vi "15-12-13 UHR-Fleezers Control (host) - 15.2.1UCB Darwin.vi"() -> ()   [LabVIEW 2014] (continued)
        n372 = stacked-sequence {
          tunnel: [w623] -> w618
          tunnel: w620 -> [w623]
          tunnel: w619 -> [w622]
          tunnel: [w622] -> w613
          frame #0 {
            n373 = Wait (ms)(milliseconds to wait=50) -> ()  [unwired: 1 out]
          }
        }
        n374 = property class="Instr"(reference=w618, error in=w613) -> (reference out=w617:refnum<visa-resource-name>, error out=w615:errorcluster, "Serial Settings:Number of Bytes at Serial Port"=w616:u32)
        "Serial Settings:Number of Bytes at Serial Port" <- w616
        n375 = VISA Read(VISA resource name=w617, byte count=w616, error in (no error)=w615) -> (read buffer=w614:string)  [unwired: 3 out]
        "read buffer" <- w614
        n376 = Fract/Exp String To Number(string=w614) -> ()  [unwired: 5 out]
      }
      event "+z", "-z": Value Change {
        n377 = event-data() -> ()  [unwired: 1 in, 5 out]
        n378 = flat-sequence {
          tunnel: w624 -> [w646]
          tunnel: w625 -> [w626]
          frame #0 {
            n379 = call "Read Stage Position.vi"("error in"=w646, "VISA resource name in"=w626) -> ("Current Position"=w631:cluster{dbl, dbl, dbl}, "error out"=w644:errorcluster, "VISA resource name out"=w645:refnum<visa-resource-name>)  [unwired: 1 out]
            n380 = local read "Saved Stage Positions"() -> (w655:dbl[][])
            n381 = Divide(x="z nudge increment (um)", y=1000.0) -> (x/y=w643:dbl)
            n382 = Boolean To (0,1)(Boolean="+z") -> (0, 1=w635:i16)
            n383 = Boolean To (0,1)(Boolean="-z") -> (0, 1=w636:i16)
            n384 = Array Subset(array=w655, index (row)=1 ("index"), length (row)=1 ("length"), index (col)=1 ("index"), length (col)=3 ("length")) -> (w652:dbl[][])
            n385 = Multiply(x=w635, y=w643) -> (x*y=w639:dbl)
            n386 = Multiply(x=w636, y=w643) -> (x*y=w637:dbl)
            n387 = Unbundle(w631) -> (w629:dbl, w628:dbl, w632:dbl)
            n388 = Negate(x=w637) -> (-x=w638:dbl)
            n389 = Reshape Array(w652, 3 ("dimension size")) -> (w650:dbl[])
            n390 = Add(x=w639, y=w638) -> (x+y=w640:dbl)
            n391 = Array To Cluster(array=w650) -> ()  [unwired: 1 out]
            n392 = Add(x=w640, y=w632) -> (x+y=w630:dbl)
            n393 = Bundle(cluster=w631, w629, w628, w630) -> (w627:cluster{dbl, dbl, dbl})
            n394 = call "Set Stage Position.vi"("Position"=w627, "error in"=w644, "VISA resource name in"=w645) -> ("error out"=w649:errorcluster)  [unwired: 2 out]
            n395 = local write "Stage Moving"(TRUE ("Stage Moving")) -> ()
            n396 = local write "Stage Control Serial Error"(w649) -> ()
          }
          frame #1 {
            n397 = local write "Stage Moving"(FALSE ("Stage Moving")) -> ()
          }
        }
      }
      event "-y", "+y": Value Change {
        n398 = event-data() -> ()  [unwired: 1 in, 5 out]
        n399 = flat-sequence {
          tunnel: w658 -> [w682]
          tunnel: w659 -> [w665]
          frame #0 {
            n400 = call "Read Stage Position.vi"("error in"=w682, "VISA resource name in"=w665) -> ("Current Position"=w668:cluster{dbl, dbl, dbl}, "error out"=w680:errorcluster, "VISA resource name out"=w681:refnum<visa-resource-name>)  [unwired: 1 out]
            n401 = Divide(x="y nudge increment (um", y=1000.0) -> (x/y=w679:dbl)
            n402 = Boolean To (0,1)(Boolean="+y") -> (0, 1=w671:i16)
            n403 = Boolean To (0,1)(Boolean="-y") -> (0, 1=w672:i16)
            n404 = Multiply(x=w671, y=w679) -> (x*y=w675:dbl)
            n405 = Multiply(x=w672, y=w679) -> (x*y=w673:dbl)
            n406 = Unbundle(w668) -> (w667:dbl, w662:dbl, w664:dbl)
            n407 = Negate(x=w673) -> (-x=w674:dbl)
            n408 = Add(x=w675, y=w674) -> (x+y=w676:dbl)
            n409 = Add(x=w676, y=w662) -> (x+y=w663:dbl)
            n410 = Bundle(cluster=w668, w667, w663, w664) -> (w666:cluster{dbl, dbl, dbl})
            n411 = call "Set Stage Position.vi"("Position"=w666, "error in"=w680, "VISA resource name in"=w681) -> ("error out"=w661:errorcluster)  [unwired: 2 out]
            n412 = local write "Stage Control Serial Error"(w661) -> ()
            n413 = local write "Stage Moving"(TRUE ("Stage Moving")) -> ()
          }
          frame #1 {
            n414 = local write "Stage Moving"(FALSE ("Stage Moving")) -> ()
          }
        }
      }
      event "-x", "+x": Value Change {
        n415 = event-data() -> ()  [unwired: 1 in, 5 out]
        n416 = flat-sequence {
          tunnel: w684 -> [w708]
          tunnel: w685 -> [w692]
          frame #0 {
            n417 = call "Read Stage Position.vi"("error in"=w708, "VISA resource name in"=w692) -> ("Current Position"=w694:cluster{dbl, dbl, dbl}, "error out"=w706:errorcluster, "VISA resource name out"=w707:refnum<visa-resource-name>)  [unwired: 1 out]
            n418 = Divide(x="x nudge increment (um)", y=1000.0) -> (x/y=w705:dbl)
            n419 = Boolean To (0,1)(Boolean="+x") -> (0, 1=w697:i16)
            n420 = Boolean To (0,1)(Boolean="-x") -> (0, 1=w698:i16)
            n421 = Multiply(x=w697, y=w705) -> (x*y=w701:dbl)
            n422 = Multiply(x=w698, y=w705) -> (x*y=w699:dbl)
            n423 = Unbundle(w694) -> (w686:dbl, w688:dbl, w691:dbl)
            n424 = Negate(x=w699) -> (-x=w700:dbl)
            n425 = Add(x=w701, y=w700) -> (x+y=w702:dbl)
            n426 = Add(x=w702, y=w686) -> (x+y=w687:dbl)
            n427 = Bundle(cluster=w694, w687, w688, w691) -> (w693:cluster{dbl, dbl, dbl})
            n428 = call "Set Stage Position.vi"("Position"=w693, "error in"=w706, "VISA resource name in"=w707) -> ("error out"=w689:errorcluster)  [unwired: 2 out]
            n429 = local write "Stage Control Serial Error"(w689) -> ()
            n430 = local write "Stage Moving"(TRUE ("Stage Moving")) -> ()
          }
          frame #1 {
            n431 = local write "Stage Moving"(FALSE ("Stage Moving")) -> ()
          }
        }
      }
      event "Cal/Data Acq. Spot": Value Change {
        n432 = event-data() -> ()  [unwired: 1 in, 5 out]
        n433 = flat-sequence {
          tunnel: w716 -> [w720]
          tunnel: w717 -> [w721]
          tunnel: [w721] -> w713
          tunnel: [w720] -> w712
          tunnel: w713 -> [w726]
          tunnel: w712 -> [w725]
          tunnel: ["Cal @ (MHz)"] -> w710
          tunnel: [w730] -> w714
          tunnel: w710 -> [w730]
          tunnel: w714 -> [w742]
          tunnel: ["W/ Offset 1"] -> w711
          tunnel: w714 -> [w763]
          tunnel: w711 -> [w761]
          frame #0 {
            n434 = property on="Sample Channel\nFlow" class="Bool (strict)"("Val(Sgnl)"="Daq spot flow on") -> ()  [unwired: 2 in, 2 out]
            n435 = Wait (ms)(milliseconds to wait=u32 250) -> ()  [unwired: 1 out]
          }
          frame #1 {
            n436 = local read "Saved Stage Positions"() -> (w723:dbl[][])
            n437 = property on="Trap Delta (MHz)" class="DigNum (strict)"("Val(Sgnl)"="Cal @ (MHz)") -> ()  [unwired: 2 in, 2 out]
            n438 = local write "Stage Moving"(TRUE ("Stage Moving")) -> ()
            n439 = call "move to saved stage position.vi"("error in"=w725, "Stage VISA resource name in"=w726, "Position"="Cal Stage Position", "Saved Stage Positions"=w723) -> ("error out"=w724:errorcluster)  [unwired: 1 out]
            n440 = local write "Stage Control Serial Error"(w724) -> ()
          }
          frame #2 {
            n441 = local write "Stage Moving"(FALSE ("Stage Moving")) -> ()
            n442 = property on="Sample Channel\nFlow" class="Bool (strict)"("Val(Sgnl)"="Flow ON during cal?") -> ()  [unwired: 2 in, 2 out]
            n443 = call <vilib>:"Beep.vi"() -> ()  [unwired: 3 in, 9 out]
          }
          frame #3 {
            n444 = Wait (ms)(milliseconds to wait=u32 1000) -> ()  [unwired: 1 out]
          }
          frame #4 {
            n445 = case shown="True" "Active cal after cal?" {
              frame False {
              }
              frame True {
                n446 = local write "Active Cal"(TRUE ("Active Cal")) -> ()
                n447 = Wait (ms)(milliseconds to wait=u32 8000) -> ()  [unwired: 1 out]
              }
            }
          }
          frame #5 {
            n448 = property on="Save Calibration" class="Bool (strict)"("Val(Sgnl)"=TRUE ("Value (Signaling)")) -> ()  [unwired: 2 in, 2 out]
          }
          frame #6 {
            n449 = Wait (ms)(milliseconds to wait=u32 2000) -> ()  [unwired: 1 out]
          }
          frame #7 {
            # "Check to see if \nsaving done"
            n450 = while {
              stop <- w738 stop-if-true
              n451 = local read "Saving..."() -> (w739:bool)
              n452 = Wait (ms)(milliseconds to wait=u32 100) -> ()  [unwired: 1 out]
              n453 = Not(x=w739) -> (.not. x?=w738:bool)
            }
          }
          frame #8 {
            n454 = case shown="True" "W/ Offset 1" {
              tunnel: w742 -> [_ w743]
              frame False {
              }
              frame True {
                n455 = stacked-sequence {
                  tunnel: w743 -> [_ _ _ _ _ _ _ w760]
                  frame #0 {
                    n456 = property on="Trap Delta (MHz)" class="DigNum (strict)"("Val(Sgnl)"="Offset 1 Start (MHz)") -> ()  [unwired: 2 in, 2 out]
                    n457 = Replace Array Subset(array=u32[] [0] ("Index Values"), new element="Offset 1 Set", index=0) -> (w744:u32[])
                    n458 = property on="Saved AOD Raster Scan Parameter Sets" class="Arr (strict)"("Index Values"=w744) -> ()  [unwired: 2 in, 2 out]
                  }
                  frame #1 {
                    n459 = Wait (ms)(milliseconds to wait=u32 200) -> ()  [unwired: 1 out]
                  }
                  frame #2 {
                    n460 = property on="Load parameters" class="Bool (strict)"("Val(Sgnl)"=TRUE ("Value (Signaling)")) -> ()  [unwired: 2 in, 2 out]
                  }
                  frame #3 {
                    n461 = Wait (ms)(milliseconds to wait=u32 200) -> ()  [unwired: 1 out]
                  }
                  frame #4 {
                    n462 = property on="Trap Raster Scan" class="Bool (strict)"("Val(Sgnl)"=TRUE ("Value (Signaling)")) -> ()  [unwired: 2 in, 2 out]
                  }
                  frame #5 {
                    n463 = Wait (ms)(milliseconds to wait=u32 2000) -> ()  [unwired: 1 out]
                  }
                  frame #6 {
                    n464 = while {
                      stop <- w757 stop-if-true
                      n465 = local read "Raster Scanning..."() -> (w759:bool)
                      n466 = local read "Saving..."() -> (w755:bool)
                      n467 = Wait (ms)(milliseconds to wait=u32 100) -> ()  [unwired: 1 out]
                      n468 = Not(x=w755) -> (.not. x?=w754:bool)
                      n469 = Not(x=w759) -> (.not. x?=w756:bool)
                      n470 = And(x=w756, y=w754) -> (x .and. y?=w757:bool)
                    }
                  }
                  frame #7 {
                    n471 = property on="Trap Delta (MHz)" class="DigNum (strict)"("Val(Sgnl)"=w760) -> ()  [unwired: 2 in, 2 out]
                  }
                }
              }
            }
          }
          frame #9 {
            n472 = local read "Save ave N"() -> (w762:dbl)
            n473 = case shown="False" "W/ Offset 2" {
              tunnel: w763 -> [_ w770]
              tunnel: w762 -> [_ w769]
              tunnel: w761 -> [w765 _]
              frame False {
                n474 = case shown="False" w765 {
                  frame False {
                    n475 = Multiply(x="Cal read wait (s)", y=u32 1000 ("milliseconds to wait")) -> (x*y=w767:u32)
                    n476 = Wait (ms)(milliseconds to wait=w767) -> ()  [unwired: 1 out]
                  }
                  frame True {
                  }
                }
              }
              frame True {
                n477 = stacked-sequence {
                  tunnel: w770 -> [_ _ _ _ _ _ _ _ _ w791 _ _]
                  tunnel: w769 -> [_ _ _ _ _ _ _ _ _ w789 _ _]
                  frame #0 {
                    n478 = property on="Save ave N" class="DigNum (strict)"("Val(Sgnl)"=1.0 ("Value (Signaling)")) -> ()  [unwired: 2 in, 2 out]
                  }
                  frame #1 {
                    n479 = Wait (ms)(milliseconds to wait=u32 500) -> ()  [unwired: 1 out]
                  }
                  frame #2 {
                    n480 = property on="Trap Delta (MHz)" class="DigNum (strict)"("Val(Sgnl)"="Offset 2 Start (MHz)") -> ()  [unwired: 2 in, 2 out]
                    n481 = Replace Array Subset(array=u32[] [0] ("Index Values"), new element="Offset 2 Set", index=0) -> (w775:u32[])
                    n482 = property on="Saved AOD Raster Scan Parameter Sets" class="Arr (strict)"("Index Values"=w775) -> ()  [unwired: 2 in, 2 out]
                  }
                  frame #3 {
                    n483 = Wait (ms)(milliseconds to wait=u32 500) -> ()  [unwired: 1 out]
                  }
                  frame #4 {
                    n484 = property on="Load parameters" class="Bool (strict)"("Val(Sgnl)"=TRUE ("Value (Signaling)")) -> ()  [unwired: 2 in, 2 out]
                  }
                  frame #5 {
                    n485 = Wait (ms)(milliseconds to wait=u32 500) -> ()  [unwired: 1 out]
                  }
                  frame #6 {
                    n486 = property on="Trap Raster Scan" class="Bool (strict)"("Val(Sgnl)"=TRUE ("Value (Signaling)")) -> ()  [unwired: 2 in, 2 out]
                  }
                  frame #7 {
                    n487 = Wait (ms)(milliseconds to wait=u32 2000) -> ()  [unwired: 1 out]
                  }
                  frame #8 {
                    n488 = while {
                      stop <- w784 stop-if-true
                      n489 = local read "Raster Scanning..."() -> (w787:bool)
                      n490 = local read "Saving..."() -> (w785:bool)
                      n491 = Wait (ms)(milliseconds to wait=u32 100) -> ()  [unwired: 1 out]
                      n492 = Not(x=w785) -> (.not. x?=w783:bool)
                      n493 = Not(x=w787) -> (.not. x?=w786:bool)
                      n494 = And(x=w786, y=w783) -> (x .and. y?=w784:bool)
                    }
                  }
                  frame #9 {
                    n495 = property on="Trap Delta (MHz)" class="DigNum (strict)"("Val(Sgnl)"=w791) -> ()  [unwired: 2 in, 2 out]
                    n496 = property on="Saved AOD Raster Scan Parameter Sets" class="Arr (strict)"("Index Values"=u32[] [0]) -> ()  [unwired: 2 in, 2 out]
                    n497 = property on="Save ave N" class="DigNum (strict)"("Val(Sgnl)"=w789) -> ()  [unwired: 2 in, 2 out]
                  }
                  frame #10 {
                    n498 = Wait (ms)(milliseconds to wait=u32 500) -> ()  [unwired: 1 out]
                  }
                  frame #11 {
                    n499 = property on="Load parameters" class="Bool (strict)"("Val(Sgnl)"=TRUE ("Value (Signaling)")) -> ()  [unwired: 2 in, 2 out]
                  }
                }
              }
            }
          }
          frame #10 {
            n500 = property on="Read Cal" class="Bool (strict)"("Val(Sgnl)"=TRUE ("Value (Signaling)")) -> ()  [unwired: 2 in, 2 out]
          }
          frame #11 {
            n501 = Wait (ms)(milliseconds to wait=u32 1000) -> ()  [unwired: 1 out]
          }
          frame #12 {
            n502 = property on="Fish for Tether" class="Bool (strict)"("Val(Sgnl)"="Fish after cal?") -> ()  [unwired: 2 in, 2 out]
          }
        }
        n503 = local write "Cal/Data Acq. Spot"(FALSE ("Cal/Data Acq. Spot")) -> ()
      }
      event "Dump Beads": Value Change {
        n504 = event-data() -> ()  [unwired: 1 in, 5 out]
        n505 = flat-sequence {
          tunnel: ["Dump spot flow on?"] -> w797
          tunnel: [w808] -> w798
          tunnel: w797 -> [w808]
          tunnel: w801 -> [w813]
          tunnel: w800 -> [w812]
          tunnel: [w810] -> w799
          tunnel: w798 -> [w810]
          tunnel: w799 -> [w823]
          frame #0 {
            w802 = FALSE ("Value (Signaling)")
            n506 = local read "Saving..."() -> (w804:bool)
            n507 = local write "Dump Beads"(FALSE ("Dump Beads")) -> ()
            n508 = property on="Inject Pump 3" class="Bool (strict)"("Val(Sgnl)"=w802) -> ()  [unwired: 2 in, 2 out]
            n509 = property on="Inject Pump 1" class="Bool (strict)"("Val(Sgnl)"=w802) -> ()  [unwired: 2 in, 2 out]
            n510 = local write "Stop Saving"(w804) -> ()
          }
          frame #1 {
            w805 = FALSE ("Fl. Triggered...")
            n511 = case shown="True" "Dump spot flow on?" {
              frame False {
              }
              frame True {
                n512 = property on="Sample Channel\nFlow" class="Bool (strict)"("Val(Sgnl)"=TRUE ("Stage Moving")) -> ()  [unwired: 2 in, 2 out]
              }
            }
            n513 = local write "Fl. Triggered..."(w805) -> ()
            n514 = local write "Tether"(w805) -> ()
            n515 = property on="Green Laser ON" class="Bool (strict)"("Val(Sgnl)"=w805) -> ()  [unwired: 2 in, 2 out]
            n516 = property on="Trap Pos. FB ON" class="Bool (strict)"("Val(Sgnl)"=w805) -> ()  [unwired: 2 in, 2 out]
            n517 = property on="Trap Trig. Fl." class="Bool (strict)"("Val(Sgnl)"=w805) -> ()  [unwired: 2 in, 2 out]
            n518 = property on="Fl. Triggered..." class="Bool (strict)"("Val(Sgnl)"=w805) -> ()  [unwired: 2 in, 2 out]
            n519 = property on="Dip for Protein" class="Bool (strict)"("Val(Sgnl)"=w805) -> ()  [unwired: 2 in, 2 out]
            n520 = property on="Pause dwell" class="Bool (strict)"("Val(Sgnl)"=w805) -> ()  [unwired: 2 in, 2 out]
          }
          frame #2 {
            n521 = property on="Trap Pos. FB Offset Factor" class="DigNum (strict)"("Val(Sgnl)"=i64 0 ("Value (Signaling)")) -> ()  [unwired: 2 in, 2 out]
          }
          frame #3 {
            n522 = local read "Saved Stage Positions"() -> (w814:dbl[][])
            n523 = local write "Stage Moving"(TRUE ("Stage Moving")) -> ()
            n524 = Array Subset(array=w814, index (row)=3 ("index"), length (row)=1 ("length"), index (col)=1 ("index"), length (col)=3 ("length")) -> (w819:dbl[][])
            n525 = Reshape Array(w819, 3 ("dimension size")) -> (w817:dbl[])
            n526 = Array To Cluster(array=w817) -> (cluster=w816:cluster{"[0]":dbl, "[1]":dbl, "[2]":dbl})
            n527 = call "Set Stage Position.vi"("Position"=w816, "error in"=w812, "VISA resource name in"=w813) -> ()  [unwired: 3 out]
          }
          frame #4 {
            w824 = FALSE ("Value (Signaling)")
            n528 = case shown="True" w823 {
              frame False {
              }
              frame True {
                n529 = property on="Sample Channel\nFlow" class="Bool (strict)"("Val(Sgnl)"=FALSE ("Stage Moving")) -> ()  [unwired: 2 in, 2 out]
              }
            }
            n530 = property on="Trap 1 (ON/OFF)" class="Bool (strict)"("Val(Sgnl)"=w824) -> ()  [unwired: 2 in, 2 out]
            n531 = property on="Trap 2 (ON/OFF)" class="Bool (strict)"("Val(Sgnl)"=w824) -> ()  [unwired: 2 in, 2 out]
            n532 = call <vilib>:"Beep.vi"() -> ()  [unwired: 3 in, 9 out]
          }
          frame #5 {
            n533 = property on="Move Cap. 2 (ADig Top)" class="Bool (strict)"("Val(Sgnl)"=TRUE ("Value (Signaling)")) -> ()  [unwired: 2 in, 2 out]
            n534 = property on="Tab Control" class="TabCtl (strict)"("Val(Sgnl)"=T30."Status" ("Value (Signaling)")) -> ()  [unwired: 2 in, 2 out]
          }
        }
      }
      event "Dip for Protein": Value Change {
        n535 = event-data() -> ()  [unwired: 1 in, 5 out]
        n536 = case shown="True" "Dip for Protein" {
          tunnel: w830 -> [_ w832]
          tunnel: w829 -> [_ w831]
          frame False {
          }
          frame True {
            n537 = while {
              tunnel: w832 -> [w843]
              tunnel: w831 -> [w842]
              i -> [w837]
              stop <- w839 stop-if-true
              n538 = Increment(x=w837) -> (x+1=→"Dip #":i32)
              n539 = flat-sequence {
                tunnel: w842 -> [w854]
                tunnel: w843 -> [w855]
                tunnel: [w855] -> w847
                tunnel: [w854] -> w846
                tunnel: [w848] -> w833
                tunnel: [w860] -> w841
                tunnel: [w861] -> w840
                tunnel: w847 -> [w862]
                tunnel: w846 -> [w863]
                tunnel: [w858] -> w834
                tunnel: w833 -> [w858]
                tunnel: [w871] -> w845
                tunnel: w841 -> [w871]
                tunnel: [w870] -> w844
                tunnel: w840 -> [w870]
                tunnel: [w867] -> w838
                tunnel: [w866] -> w835
                tunnel: w834 -> [w866]
                tunnel: w844 -> [w891]
                tunnel: w845 -> [w892]
                tunnel: w838 -> [w893]
                tunnel: w835 -> [w890]
                tunnel: [w949] -> w839
                frame #0 {
                  n540 = local read "Trap Pos. FB ON"() -> (w848:bool)
                  n541 = Compound Arithmetic op=AND("Flow ON\nduring dip?", "FB OFF when \nflow ON", w848) -> (w849:bool)
                  n542 = case shown="True" "Move trap \nbefore dip move?" {
                    frame False {
                    }
                    frame True {
                      n543 = property on="Trap Delta (MHz)" class="DigNum (strict)"("Val(Sgnl)"="Dipping Delta (MHz)") -> ()  [unwired: 2 in, 2 out]
                    }
                  }
                  n544 = property on="Green Laser ON" class="Bool (strict)"("Val(Sgnl)"="Green ON\nbefore dip?") -> ()  [unwired: 2 in, 2 out]
                  n545 = property on="Sample Channel\nFlow" class="Bool (strict)"("Val(Sgnl)"="Flow ON\nduring dip?") -> ()  [unwired: 2 in, 2 out]
                  n546 = case shown="True" w849 {
                    frame False {
                    }
                    frame True {
                      n547 = property on="Trap Pos. FB ON" class="Bool (strict)"("Val(Sgnl)"=FALSE ("Value (Signaling)")) -> ()  [unwired: 2 in, 2 out]
                    }
                  }
                }
                frame #1 {
                  n548 = local read "Saved Stage Positions"() -> (w865:dbl[][])
                  n549 = local write "Cancel dwell"(FALSE ("Cancel dwell")) -> ()
                  n550 = call "move to saved stage position.vi"("error in"=w863, "Stage VISA resource name in"=w862, "Position"="Dip Stage \nPosition", "Saved Stage Positions"=w865) -> ("VISA resource name out"=w860:refnum<visa-resource-name>, "error out"=w861:errorcluster)
                }
                frame #2 {
                  n551 = node-c288() -> (w869:T27)  [unwired: 4 in]
                  n552 = timed-loop {
                    timing: w869 -> [_]
                    timing-out: [_] -> w868
                    tunnel: [w875] -> w867
                    i -> [w872]
                    stop <- w876 stop-if-true
                    n553 = node-c288() -> ()  [unwired: 1 in, 1 out]
                    n554 = Greater Or Equal?(x=w872, y="Dip Duration (s)") -> (x >= y?=w884:bool)
                    n555 = local read "Dip for Protein"() -> (w877:bool)
                    n556 = local read "Dump Beads"() -> (w874:bool)
                    n557 = local read "Cancel dwell"() -> (w883:bool)
                    n558 = local read "Pause dwell"() -> (w880:bool)
                    n559 = Not(x=w877) -> (.not. x?=w882:bool)
                    n560 = Compound Arithmetic op=OR(w883, w884, w882) -> (w881:bool)
                    n561 = Select(t=FALSE, s=w880, f=w881) -> (s? t:f=w878:bool)
                    n562 = Not(x=w874) -> (.not. x?=w873:bool)
                    n563 = node-c288() -> ()  [unwired: 1 in, 1 out]
                    n564 = And(x=w877, y=w873) -> (x .and. y?=w875:bool)
                    n565 = Or(x=w878, y=w874) -> (x .or. y?=w876:bool)
                    "Dip Time (s)" <- w872
                  }
                  n566 = node-c288(w868) -> ()  [unwired: 1 out]
                }
                frame #3 {
                  n567 = case shown="True" w893 {
                    tunnel: w892 -> [_ w898]
                    tunnel: w891 -> [_ w897]
                    tunnel: w890 -> [_ w894]
                    frame False {
                    }
                    frame True {
                      n568 = flat-sequence {
                        tunnel: w897 -> [w902]
                        tunnel: w898 -> [w903]
                        tunnel: [w903] -> w896
                        tunnel: [w902] -> w895
                        tunnel: w894 -> [w899]
                        tunnel: w896 -> [w913]
                        tunnel: w895 -> [w912]
                        tunnel: w894 -> [w921]
                        frame #0 {
                          n569 = local read "Sample Channel\nFlow"() -> (w901:bool)
                          n570 = case shown="True" w901 {
                            tunnel: "Flow ON \nduring return\nfrom dip?" -> [w904 w907]
                            tunnel: w899 -> [_ w906]
                            frame False {
                              n571 = case shown="True" w904 {
                                frame False {
                                }
                                frame True {
                                n572 = property on="Sample Channel\nFlow" class="Bool (strict)"("Val(Sgnl)"=TRUE ("Value (Signaling)")) -> ()  [unwired: 2 in, 2 out]
                                }
                              }
                            }
                            frame True {
                              n573 = case shown="False" w907 {
                                tunnel: w906 -> [w908 _]
                                frame False {
                                n574 = property on="Trap Pos. FB ON" class="Bool (strict)"("Val(Sgnl)"=w908) -> ()  [unwired: 2 in, 2 out]
                                n575 = property on="Sample Channel\nFlow" class="Bool (strict)"("Val(Sgnl)"=FALSE ("Value (Signaling)")) -> ()  [unwired: 2 in, 2 out]
                                }
                                frame True {
                                }
                              }
                            }
                          }
                        }
                        frame #1 {
                          # "For turning on green laser before stage reaches lower spot"
                          n576 = case shown="True" "Green ON\nafter start\nreturn?" {
                            frame False {
                            }
                            frame True {
                              n577 = flat-sequence {
                                frame #0 {
                                n578 = Multiply(x="Green delay after \nstart return (s)", y=1000.0) -> (x*y=w918:dbl)
                                n579 = Wait (ms)(milliseconds to wait=w918) -> ()  [unwired: 1 out]
                                }
                                frame #1 {
                                n580 = property on="Green Laser ON" class="Bool (strict)"("Val(Sgnl)"=TRUE ("Value (Signaling)")) -> ()  [unwired: 2 in, 2 out]
                                }
                              }
                            }
                          }
                          n581 = local read "Saved Stage Positions"() -> (w916:dbl[][])
                          n582 = local write "Cancel dwell"(FALSE ("Cancel dwell")) -> ()
                          n583 = call "move to saved stage position.vi"("error in"=w912, "Stage VISA resource name in"=w913, "Position"="Return Stage \nPosition", "Saved Stage Positions"=w916) -> ("error out"=w914:errorcluster)  [unwired: 1 out]
                          n584 = local write "Stage Control Serial Error"(w914) -> ()
                        }
                        frame #2 {
                          n585 = property on="Trap Pos. FB ON" class="Bool (strict)"("Val(Sgnl)"=w921) -> ()  [unwired: 2 in, 2 out]
                          n586 = case shown="True" "Green ON \nafter return?" {
                            frame False {
                            }
                            frame True {
                              n587 = property on="Green Laser ON" class="Bool (strict)"("Val(Sgnl)"=TRUE ("Value (Signaling)")) -> ()  [unwired: 2 in, 2 out]
                            }
                          }
                          n588 = case shown="True" "Move trap after return?" {
                            frame False {
                            }
                            frame True {
                              n589 = property on="Trap Delta (MHz)" class="DigNum (strict)"("Val(Sgnl)"="Dip Trap Delta 2 (MHz)") -> ()  [unwired: 2 in, 2 out]
                            }
                          }
                          n590 = case shown="True" "Save data after return?" {
                            frame False {
                            }
                            frame True {
                              n591 = property on="Start Saving" class="Bool (strict)"("Val(Sgnl)"=TRUE ("Value (Signaling)")) -> ()  [unwired: 2 in, 2 out]
                            }
                          }
                          n592 = property on="Sample Channel\nFlow" class="Bool (strict)"("Val(Sgnl)"="Flow ON\nduring daq?") -> ()  [unwired: 2 in, 2 out]
                        }
                        frame #3 {
                          n593 = node-c288() -> (w930:T27)  [unwired: 4 in]
                          n594 = timed-loop {
                            timing: w930 -> [_]
                            timing-out: [_] -> w929
                            i -> [w931]
                            stop <- w933 stop-if-true
                            n595 = node-c288() -> ()  [unwired: 1 in, 1 out]
                            n596 = local read "Dump Beads"() -> (w932:bool)
                            n597 = Greater Or Equal?(x=w931, y="Dwell Duration (s)") -> (x >= y?=w938:bool)
                            n598 = local read "Dip for Protein"() -> (w935:bool)
                            n599 = Not(x=w935) -> (.not. x?=w934:bool)
                            n600 = Compound Arithmetic op=OR(w938, "Cancel dwell", w934) -> (w937:bool)
                            n601 = node-c288() -> ()  [unwired: 1 in, 1 out]
                            n602 = Select(t=FALSE, s="Pause dwell", f=w937) -> (s? t:f=w940:bool)
                            n603 = Or(x=w940, y=w932) -> (x .or. y?=w933:bool)
                            "Dwell Time (s)" <- w931
                          }
                          n604 = node-c288(w929) -> ()  [unwired: 1 out]
                        }
                      }
                    }
                  }
                }
                frame #4 {
                  n605 = local read "Dip for Protein"() -> (w950:bool)
                  n606 = local read "Dump Beads"() -> (w947:bool)
                  n607 = local write "Cancel dwell"(FALSE ("Cancel dwell")) -> ()
                  n608 = Not(x=w950) -> (.not. x?=w951:bool)
                  n609 = Not(x="Cont. Repeat Dipping?") -> (.not. x?=w953:bool)
                  n610 = Compound Arithmetic op=OR(w951, w953, w947) -> (w949:bool)
                }
              }
            }
          }
        }
      }
      event "Profile": Value Change {
        n611 = event-data() -> ()  [unwired: 1 in, 5 out]
        n612 = flat-sequence {
          tunnel: w962 -> [w965]
          tunnel: w961 -> [w973]
          tunnel: [w967] -> w960
          tunnel: [w966] -> w959
          tunnel: [w964] -> w957
          tunnel: [w963] -> w954
          tunnel: w960 -> [w980]
          tunnel: w959 -> [w979]
          tunnel: [w977] -> w958
          tunnel: w957 -> [w978]
          tunnel: [w976] -> w956
          tunnel: [w975] -> w955
          tunnel: w954 -> [w975]
          tunnel: w958 -> [w984]
          tunnel: w956 -> [w983]
          tunnel: w955 -> [w982]
          frame #0 {
            n613 = call "Read Stage Position.vi"("error in"=w973, "VISA resource name in"=w965) -> ("Current Position"=w963:cluster{dbl, dbl, dbl}, "error out"=w966:errorcluster, "VISA resource name out"=w964:refnum<visa-resource-name>)  [unwired: 1 out]
            "Current Position" <- w963
            n614 = local write "Stage Control Serial Error"(w966) -> ()
            n615 = Unbundle(w963) -> (w970:dbl, w972:dbl, w968:dbl)
            n616 = Add(x=w972, y="Y change (mm)") -> (x+y=w969:dbl)
            n617 = Bundle(w970, w969, w968) -> (w967:cluster{dbl, dbl, dbl})  [unwired: 1 in]
          }
          frame #1 {
            # "move to new position and start saving"
            n618 = local write "Stage Moving"(TRUE ("Stage Moving")) -> ()
            n619 = local write "Start Saving"(TRUE ("Start Saving")) -> ()
            n620 = call "Set Stage Position.vi"("Position"=w980, "error in"=w979, "VISA resource name in"=w978) -> ("error out"=w976:errorcluster, "VISA resource name out"=w977:refnum<visa-resource-name>)  [unwired: 1 out]
          }
          frame #2 {
            # "go back to start"
            n621 = call "Set Stage Position.vi"("Position"=w982, "error in"=w983, "VISA resource name in"=w984) -> ()  [unwired: 3 out]
          }
          frame #3 {
            # "stop saving"
            n622 = local write "Stop Saving"(TRUE ("Stop Saving")) -> ()
            n623 = local write "Stage Moving"(FALSE ("Stage Moving")) -> ()
          }
        }
      }
      event "Move to Position 1", "Move to Position 2", "Move to Position 3", "Move to Position 4", "Move to Position 5", "Lower Ch. Cap.", "Move to Position 6": Value Change {
        n624 = event-data() -> ()  [unwired: 1 in, 5 out]
        n625 = Or(x="Move to Position 5", y="Lower Ch. Cap.") -> (x .or. y?=w991:bool)
        n626 = Build Array("Move to Position 1", "Move to Position 2", "Move to Position 3", "Move to Position 4", w991, "Move to Position 6") -> (w994:bool[])
        n627 = Boolean Array To Number(Boolean array=w994) -> (number=w993:u32)
        n628 = Logarithm Base 2(1:w993) -> (0:w992:dbl)
        n629 = flat-sequence {
          tunnel: w992 -> [w1003]
          tunnel: w989 -> [w1001]
          tunnel: w988 -> [w1000]
          frame #0 {
            n630 = local read "Saved Stage Positions"() -> (w1011:dbl[][])
            n631 = Array Subset(array=w1011, index (row)=w1003, length (row)=1 ("length"), index (col)=1 ("index"), length (col)=3 ("length")) -> (w1008:dbl[][])
            n632 = Reshape Array(w1008, 3 ("dimension size")) -> (w1006:dbl[])
            n633 = Array To Cluster(array=w1006) -> (cluster=w1005:cluster{"[0]":dbl, "[1]":dbl, "[2]":dbl})
            n634 = call "Set Stage Position.vi"("Position"=w1005, "error in"=w1000, "VISA resource name in"=w1001) -> ("error out"=w1004:errorcluster)  [unwired: 2 out]
            n635 = local write "Stage Moving"(TRUE ("Stage Moving")) -> ()
            n636 = local write "Stage Control Serial Error"(w1004) -> ()
          }
          frame #1 {
            n637 = local write "Stage Moving"(FALSE ("Stage Moving")) -> ()
            n638 = call <vilib>:"Beep.vi"() -> ()  [unwired: 3 in, 9 out]
          }
        }
      }
      event "Got ADig bead": Value Change {
        n639 = event-data() -> ()  [unwired: 1 in, 5 out]
        n640 = flat-sequence {
          frame #0 {
            n641 = local read "Cap 1 Samp Flow ON"() -> (w1015:bool)
            n642 = case shown="True" w1015 {
              frame False {
              }
              frame True {
                n643 = property on="Sample Channel\nFlow" class="Bool (strict)"("Val(Sgnl)"=TRUE ("Value (Signaling)")) -> ()  [unwired: 2 in, 2 out]
              }
            }
          }
          frame #1 {
            n644 = property on="Inject Pump 3" class="Bool (strict)"("Val(Sgnl)"=FALSE ("Value (Signaling)")) -> ()  [unwired: 2 in, 2 out]
          }
          frame #2 {
            n645 = property on="Move Cap. 1 (DNA Bottom)" class="Bool (strict)"("Val(Sgnl)"=TRUE ("Value (Signaling)")) -> ()  [unwired: 2 in, 2 out]
          }
        }
      }
      event "Force FB Data\nScript": Value Change {
        n646 = event-data() -> ()  [unwired: 1 in, 5 out]
        n647 = flat-sequence {
          tunnel: w1024 -> [w1028]
          tunnel: w1025 -> [w1029]
          tunnel: [w1029] -> w1020
          tunnel: [w1028] -> w1019
          tunnel: w1020 -> [w1032]
          tunnel: w1019 -> [w1031]
          tunnel: ["Trap Trig Fl."] -> w1021
          tunnel: [w1057] -> w1022
          tunnel: w1021 -> [w1057]
          tunnel: [w1061] -> w1023
          tunnel: w1022 -> [w1061]
          tunnel: w1023 -> [w1063]
          frame #0 {
            n648 = property on="Trap Delta (MHz)" class="DigNum (strict)"("Val(Sgnl)"="Trap Delta Before Moving") -> ()  [unwired: 2 in, 2 out]
          }
          frame #1 {
            n649 = local read "Saved Stage Positions"() -> (w1034:dbl[][])
            n650 = property on="Trap Pos. FB Offset Factor" class="DigNum (strict)"("Val(Sgnl)"=i64 0 ("Value (Signaling)")) -> ()  [unwired: 2 in, 2 out]
            n651 = local write "FB Trap Pos Offset"(0.0 ("FB Trap Pos Offset")) -> ()
            n652 = local write "Stage Moving"(TRUE ("Stage Moving")) -> ()
            n653 = call "move to saved stage position.vi"("error in"=w1031, "Stage VISA resource name in"=w1032, "Position"="Stage Position To Establish FB", "Saved Stage Positions"=w1034) -> ("error out"=w1030:errorcluster)  [unwired: 1 out]
            n654 = local write "Stage Control Serial Error"(w1030) -> ()
          }
          frame #2 {
            n655 = call <vilib>:"Beep.vi"() -> ()  [unwired: 3 in, 9 out]
            n656 = Multiply(x="Wait (s)", y=u32 1000 ("milliseconds to wait")) -> (x*y=w1041:u32)
            n657 = property on="Trap Delta (MHz)" class="DigNum (strict)"("Val(Sgnl)"="Starting \nTrap Delta (MHz)") -> ()  [unwired: 2 in, 2 out]
            n658 = local write "Stage Moving"(FALSE ("Stage Moving")) -> ()
            n659 = Wait (ms)(milliseconds to wait=w1041) -> ()  [unwired: 1 out]
            n660 = property on="Tab Control 2" class="TabCtl (strict)"("Val(Sgnl)"=T8."Feedback on Trap Position" ("Value (Signaling)")) -> ()  [unwired: 2 in, 2 out]
            n661 = property on="Tab Control" class="TabCtl (strict)"("Val(Sgnl)"=T31."Trap Control (RF)" ("Value (Signaling)")) -> ()  [unwired: 2 in, 2 out]
          }
          frame #3 {
            n662 = property on="Set Reading to\nSetpoint" class="Bool (strict)"("Val(Sgnl)"=TRUE ("Value (Signaling)")) -> ()  [unwired: 2 in, 2 out]
            n663 = Wait (ms)(milliseconds to wait=u32 500) -> ()  [unwired: 1 out]
          }
          frame #4 {
            n664 = property on="Trap Pos. FB ON" class="Bool (strict)"("Val(Sgnl)"=TRUE ("Value (Signaling)")) -> ()  [unwired: 2 in, 2 out]
            n665 = Wait (ms)(milliseconds to wait=u32 250) -> ()  [unwired: 1 out]
          }
          frame #5 {
            n666 = case shown="False" "Trap Trig Fl." {
              frame False {
                n667 = case shown="True" "Green ON after FB ON?" {
                  selector: "Green ON after FB ON?" -> [_ w1056]
                  frame False {
                  }
                  frame True {
                    n668 = property on="Green Laser ON" class="Bool (strict)"("Val(Sgnl)"=w1056) -> ()  [unwired: 2 in, 2 out]
                  }
                }
              }
              frame True {
              }
            }
            n669 = case shown="True" "Remove Action Offset" {
              tunnel: TRUE ("Value (Signaling)") -> [w1053 w1054]
              frame False {
                n670 = property on="Remove Unwinding Offset" class="Bool (strict)"("Val(Sgnl)"=w1053) -> ()  [unwired: 2 in, 2 out]
              }
              frame True {
                n671 = property on="Remove Action Offset" class="Bool (strict)"("Val(Sgnl)"=w1054) -> ()  [unwired: 2 in, 2 out]
              }
            }
            n672 = Wait (ms)(milliseconds to wait=u32 250) -> ()  [unwired: 1 out]
          }
          frame #6 {
            n673 = property on="Start Saving" class="Bool (strict)"("Val(Sgnl)"=TRUE ("Value (Signaling)")) -> ()  [unwired: 2 in, 2 out]
            n674 = Wait (ms)(milliseconds to wait=u32 5000) -> ()  [unwired: 1 out]
          }
          frame #7 {
            w1060 = TRUE ("Value (Signaling)")
            n675 = property on="Rem fb disp offset" class="Bool (strict)"("Val(Sgnl)"=w1060) -> ()  [unwired: 2 in, 2 out]
            n676 = property on="Remove Offset" class="Bool (strict)"("Val(Sgnl)"=w1060) -> ()  [unwired: 2 in, 2 out]
            n677 = Wait (ms)(milliseconds to wait=u32 100) -> ()  [unwired: 1 out]
          }
          frame #8 {
            n678 = case shown="True" w1063 {
              frame False {
              }
              frame True {
                n679 = local write "Trap Trig. Fl."(TRUE ("Value (Signaling)")) -> ()
              }
            }
          }
          frame #9 {
            n680 = case shown="True" "Start dipping after?" {
              frame False {
              }
              frame True {
                n681 = flat-sequence {
                  frame #0 {
                    n682 = Multiply(x="Delay before dipping (s)", y=1000.0) -> (x*y=w1067:dbl)
                    n683 = Wait (ms)(milliseconds to wait=w1067) -> ()  [unwired: 1 out]
                  }
                  frame #1 {
                    n684 = property on="Dip for Protein" class="Bool (strict)"("Val(Sgnl)"=TRUE ("Value (Signaling)")) -> ()  [unwired: 2 in, 2 out]
                    n685 = local write "Scripts"(T1."Dipping" ("Scripts")) -> ()
                  }
                }
              }
            }
          }
        }
      }
      event "Fixed Traps Data\nScript": Value Change {
        n686 = event-data() -> ()  [unwired: 1 in, 5 out]
        n687 = flat-sequence {
          frame #0 {
            n688 = case shown="True" "Green ON" {
              frame False {
              }
              frame True {
                n689 = property on="Green Laser ON" class="Bool (strict)"("Val(Sgnl)"=TRUE) -> ()  [unwired: 2 in, 2 out]
              }
            }
            n690 = local write "Offset (nm)"(0.0 ("Offset (nm)")) -> ()
            n691 = property on="Sample Channel\nFlow" class="Bool (strict)"("Val(Sgnl)"=FALSE ("Value (Signaling)")) -> ()  [unwired: 2 in, 2 out]
            n692 = property on="Trap Delta (MHz)" class="DigNum (strict)"("Val(Sgnl)"="Fixed Traps Trap Delta (MHz)") -> ()  [unwired: 2 in, 2 out]
          }
          frame #1 {
            n693 = Wait (ms)(milliseconds to wait=u32 1000) -> ()  [unwired: 1 out]
          }
          frame #2 {
            n694 = local write "Start Saving"(TRUE ("Start Saving")) -> ()
          }
          frame #3 {
            n695 = local read "Bead Sep. Int. Time (s)"() -> (w1078:dbl)
            n696 = Multiply(x=w1078, y=1000.0) -> (x*y=w1080:dbl)
            n697 = Wait (ms)(milliseconds to wait=w1080) -> ()  [unwired: 1 out]
          }
          frame #4 {
            n698 = property on="Remove Offset" class="Bool (strict)"("Val(Sgnl)"=TRUE ("Value (Signaling)")) -> ()  [unwired: 2 in, 2 out]
          }
          frame #5 {
            n699 = property on="Dip for Protein" class="Bool (strict)"("Val(Sgnl)"="Start dipping after?") -> ()  [unwired: 2 in, 2 out]
          }
        }
      }
      event "Got DNA bead": Value Change {
        n700 = event-data() -> ()  [unwired: 1 in, 5 out]
        n701 = flat-sequence {
          frame #0 {
            n702 = local read "Daq spot flow on"() -> (w1085:bool)
            n703 = case shown="True" w1085 {
              frame False {
              }
              frame True {
                n704 = property on="Sample Channel\nFlow" class="Bool (strict)"("Val(Sgnl)"=TRUE ("Value (Signaling)")) -> ()  [unwired: 2 in, 2 out]
              }
            }
            n705 = property on="Got DNA bead" class="Bool"("Key Focus"=FALSE) -> ()  [unwired: 2 in, 2 out]
          }
          frame #1 {
            n706 = property on="Inject Pump 1" class="Bool (strict)"("Val(Sgnl)"=FALSE ("Value (Signaling)")) -> ()  [unwired: 2 in, 2 out]
          }
          frame #2 {
            n707 = property on="Cal/Data Acq. Spot" class="Bool (strict)"("Val(Sgnl)"=TRUE ("Value (Signaling)")) -> ()  [unwired: 2 in, 2 out]
          }
        }
      }
      event "Take Stepping Data": Value Change {
        n708 = event-data() -> ()  [unwired: 1 in, 5 out]
        n709 = local read "Save ave N"() -> (w1097:dbl)
        n710 = flat-sequence {
          tunnel: w1097 -> [w1099]
          tunnel: [w1099] -> w1092
          tunnel: [w1101] -> w1093
          tunnel: w1092 -> [w1101]
          tunnel: [w1103] -> w1094
          tunnel: w1093 -> [w1103]
          tunnel: [w1106] -> w1095
          tunnel: w1094 -> [w1106]
          tunnel: [w1108] -> w1096
          tunnel: w1095 -> [w1108]
          tunnel: [w1110] -> w1090
          tunnel: w1096 -> [w1110]
          tunnel: w1090 -> [w1113]
          tunnel: [w1113] -> w1089
          tunnel: w1089 -> [w1114]
          tunnel: [w1114] -> w1091
          tunnel: w1091 -> [w1120]
          frame #0 {
            n711 = property on="Save ave N" class="DigNum (strict)"("Val(Sgnl)"="Save ave factor") -> ()  [unwired: 2 in, 2 out]
          }
          frame #1 {
            n712 = Wait (ms)(milliseconds to wait=u32 100) -> ()  [unwired: 1 out]
          }
          frame #2 {
            n713 = local read "Offset 2 Start (MHz)"() -> (w1105:dbl)
            n714 = property on="Saved AOD Raster Scan Parameter Sets" class="Arr (strict)"("Index Values"=u32[] [2]) -> ()  [unwired: 2 in, 2 out]
            n715 = property on="Trap Delta (MHz)" class="DigNum (strict)"("Val(Sgnl)"=w1105) -> ()  [unwired: 2 in, 2 out]
          }
          frame #3 {
            n716 = property on="Load parameters" class="Bool (strict)"("Val(Sgnl)"=TRUE ("Value (Signaling)")) -> ()  [unwired: 2 in, 2 out]
          }
          frame #4 {
            n717 = Wait (ms)(milliseconds to wait=u32 100) -> ()  [unwired: 1 out]
          }
          frame #5 {
            n718 = property on="Trap Raster Scan" class="Bool (strict)"("Val(Sgnl)"=TRUE ("Value (Signaling)")) -> ()  [unwired: 2 in, 2 out]
          }
          frame #6 {
            n719 = Wait (ms)(milliseconds to wait=u32 1000) -> ()  [unwired: 1 out]
          }
          frame #7 {
            n720 = while {
              stop <- w1117 stop-if-true
              n721 = local read "Raster Scanning..."() -> (w1119:bool)
              n722 = local read "Saving..."() -> (w1118:bool)
              n723 = Not(x=w1118) -> (.not. x?=w1115:bool)
              n724 = Not(x=w1119) -> (.not. x?=w1116:bool)
              n725 = And(x=w1116, y=w1115) -> (x .and. y?=w1117:bool)
            }
          }
          frame #8 {
            n726 = property on="Save ave N" class="DigNum (strict)"("Val(Sgnl)"=w1120) -> ()  [unwired: 2 in, 2 out]
          }
        }
      }
      event "Step Size (nm)": Value Change {
        n727 = event-data() -> ()  [unwired: 1 in, 5 out]
        n728 = flat-sequence {
          frame #0 {
            n729 = property on="Saved AOD Raster Scan Parameter Sets" class="Arr (strict)"("Index Values"=u32[] [1]) -> ()  [unwired: 2 in, 2 out]
          }
          frame #1 {
            n730 = Multiply(x="N Steps", y="Step Size (nm)") -> (x*y=w1122:dbl)
            n731 = property on="Scan Speed AOD (nm/s) 2" class="DigNum (strict)"("Value"="Step Size (nm)") -> ()  [unwired: 2 in, 2 out]
            n732 = property on="Step Size AOD (nm) 2" class="DigNum (strict)"("Value"="Step Size (nm)") -> ()  [unwired: 2 in, 2 out]
            n733 = property on="Scan Range AOD (nm) 2" class="DigNum (strict)"("Value"=w1122) -> ()  [unwired: 2 in, 2 out]
          }
        }
      }
      event "Take Detection Laser\nImage": Value Change {
        n734 = event-data() -> ()  [unwired: 1 in, 5 out]
        n735 = flat-sequence {
          tunnel: [w1150] -> w1140
          tunnel: [w1149] -> w1133
          tunnel: [w1148] -> w1125
          tunnel: [w1153] -> w1141
          tunnel: w1140 -> [w1153]
          tunnel: [w1152] -> w1134
          tunnel: w1133 -> [w1152]
          tunnel: [w1151] -> w1126
          tunnel: w1125 -> [w1151]
          tunnel: [w1157] -> w1142
          tunnel: w1141 -> [w1157]
          tunnel: [w1156] -> w1135
          tunnel: w1134 -> [w1156]
          tunnel: [w1155] -> w1127
          tunnel: w1126 -> [w1155]
          tunnel: [w1163] -> w1143
          tunnel: w1142 -> [w1163]
          tunnel: [w1162] -> w1136
          tunnel: w1135 -> [w1162]
          tunnel: [w1161] -> w1128
          tunnel: w1127 -> [w1161]
          tunnel: [w1167] -> w1144
          tunnel: w1143 -> [w1167]
          tunnel: [w1166] -> w1137
          tunnel: w1136 -> [w1166]
          tunnel: [w1165] -> w1129
          tunnel: w1128 -> [w1165]
          tunnel: [w1171] -> w1145
          tunnel: w1144 -> [w1171]
          tunnel: [w1170] -> w1138
          tunnel: w1137 -> [w1170]
          tunnel: [w1169] -> w1130
          tunnel: w1129 -> [w1169]
          tunnel: [w1175] -> w1146
          tunnel: w1145 -> [w1175]
          tunnel: [w1174] -> w1139
          tunnel: w1138 -> [w1174]
          tunnel: [w1173] -> w1131
          tunnel: w1130 -> [w1173]
          tunnel: w1146 -> [w1181]
          tunnel: w1139 -> [w1180]
          tunnel: [w1178] -> w1132
          tunnel: w1131 -> [w1178]
          tunnel: w1132 -> [w1182]
          frame #0 {
            n736 = local read "Laser interlacing mode"() -> (w1149:enum32{"Laser ON", "Laser OFF", "Interlace"})
            n737 = local read "Green FB On/Off"() -> (w1148:bool)
            n738 = local read "Green Laser ON"() -> (w1150:bool)
          }
          frame #1 {
            n739 = property on="Green FB On/Off" class="Bool (strict)"("Val(Sgnl)"=FALSE ("Value (Signaling)")) -> ()  [unwired: 2 in, 2 out]
          }
          frame #2 {
            n740 = property on="Green Laser ON" class="Bool (strict)"("Val(Sgnl)"=TRUE ("Value (Signaling)")) -> ()  [unwired: 2 in, 2 out]
            n741 = property on="Flip Green Filter" class="Bool (strict)"("Val(Sgnl)"=TRUE ("Value (Signaling)")) -> ()  [unwired: 2 in, 2 out]
            n742 = property on="Laser interlacing mode" class="RadioBtnsControl (strict)"("Val(Sgnl)"=enum32{"Laser ON", "Laser OFF", "Interlace"}."Laser ON" ("Value (Signaling)")) -> ()  [unwired: 2 in, 2 out]
          }
          frame #3 {
            n743 = Wait (ms)(milliseconds to wait=u32 500) -> ()  [unwired: 1 out]
          }
          frame #4 {
            n744 = property on="Confocal Image" class="Bool (strict)"("Val(Sgnl)"=TRUE ("Value (Signaling)")) -> ()  [unwired: 2 in, 2 out]
          }
          frame #5 {
            n745 = Wait (ms)(milliseconds to wait=u32 2000) -> ()  [unwired: 1 out]
          }
          frame #6 {
            n746 = while {
              stop <- w1176 stop-if-true
              n747 = local read "Saving..."() -> (w1177:bool)
              n748 = Not(x=w1177) -> (.not. x?=w1176:bool)
            }
          }
          frame #7 {
            n749 = property on="Flip Green Filter" class="Bool (strict)"("Val(Sgnl)"=TRUE ("Value (Signaling)")) -> ()  [unwired: 2 in, 2 out]
            n750 = property on="Green Laser ON" class="Bool (strict)"("Val(Sgnl)"=w1181) -> ()  [unwired: 2 in, 2 out]
            n751 = property on="Laser interlacing mode" class="RadioBtnsControl (strict)"("Val(Sgnl)"=w1180) -> ()  [unwired: 2 in, 2 out]
          }
          frame #8 {
            n752 = property on="Green FB On/Off" class="Bool (strict)"("Val(Sgnl)"=w1182) -> ()  [unwired: 2 in, 2 out]
          }
        }
      }
      event "Move in a Circle": Value Change {
        w1184 = dbl[] []
        # "converting distance (d) to angle (a)\na=arcsin(d/2r)"
        # "radius"
        # "radius"
        # "T1 Y"
        # "T1 X"
        n753 = event-data() -> ()  [unwired: 1 in, 5 out]
        n754 = local read "BD 1 Frequency 1 (MHz)"() -> (w1192:dbl)
        n755 = local read "BD 2 Frequency 1 (MHz)"() -> (w1191:dbl)
        n756 = local read "BD 1 Frequency 2 (MHz)"() -> (w1190:dbl)
        n757 = local read "BD 2 Frequency 2 (MHz)"() -> (w1189:dbl)
        n758 = Subtract(x=w1191, y="Center Y Frequency (MHz)") -> (x-y=w1196:dbl)
        n759 = Absolute Value(x=w1196) -> (abs(x)=w1187:dbl)
        n760 = flat-sequence {
          tunnel: w1187 -> [w1199]
          tunnel: [w1199] -> w1186
          frame #0 {
            n761 = local write "Radius (MHz)"(w1199) -> ()
          }
        }
        n762 = node-c288("Time step (ms)") -> (w1198:T27)  [unwired: 3 in]
        n763 = timed-loop {
          timing: w1198 -> [_]
          timing-out: [_] -> w1197
          tunnel: w1192 -> [w1290]
          tunnel: w1191 -> [_]
          tunnel: w1190 -> [w1294]